vi "Laser Ablation and Capture.vi"() -> ()   [LabVIEW 2016] (continued)
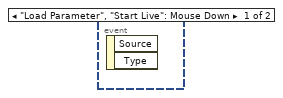
[diagram p2: hidden frame]
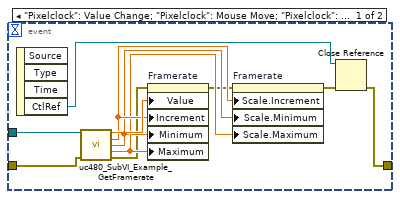
[diagram p3: hidden frame]
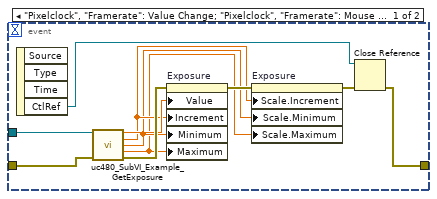
[diagram p4: hidden frame]
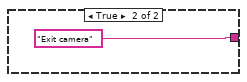
[diagram p5: hidden frame]
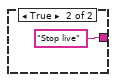
[diagram p6: hidden frame]
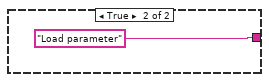
[diagram p7: hidden frame]
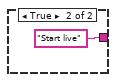
[diagram p8: hidden frame]
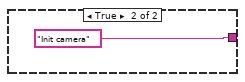
[diagram p9: hidden frame]
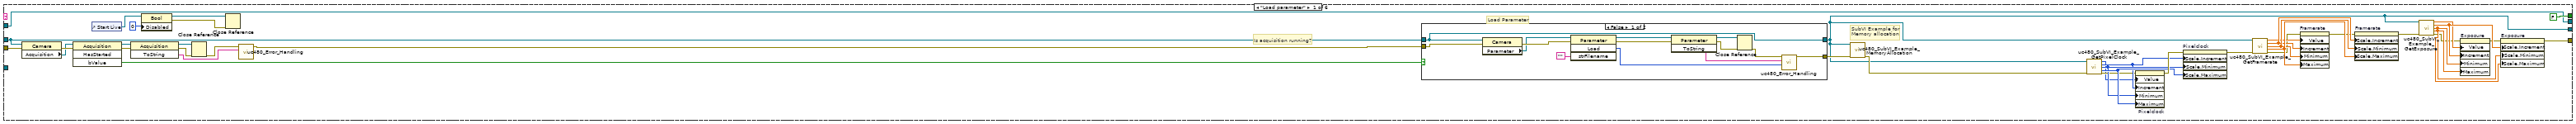
[diagram p10: hidden frame]
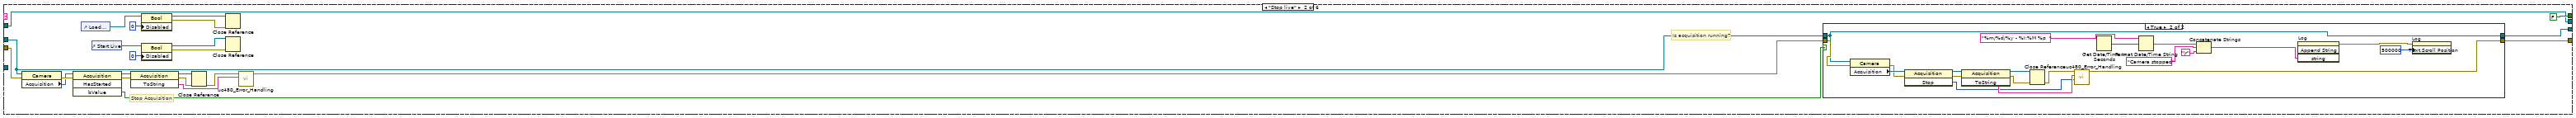
[diagram p12: hidden frame]
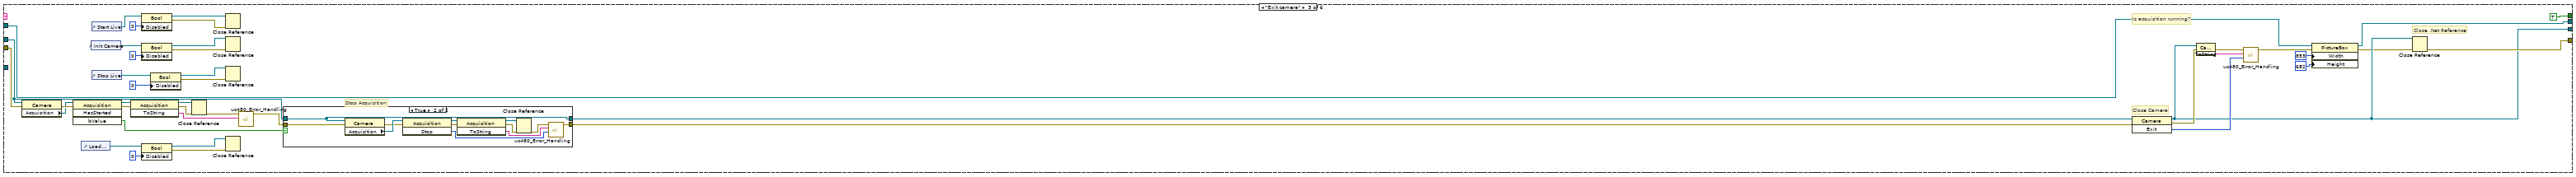
[diagram p14: hidden frame]
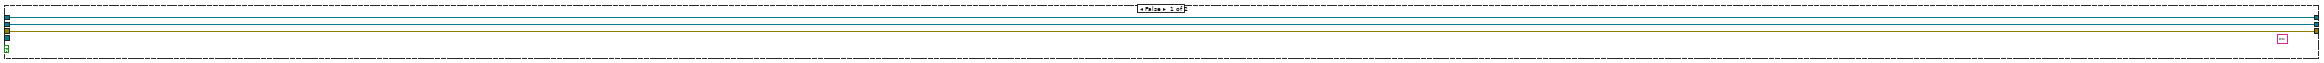
[diagram p16: hidden frame]
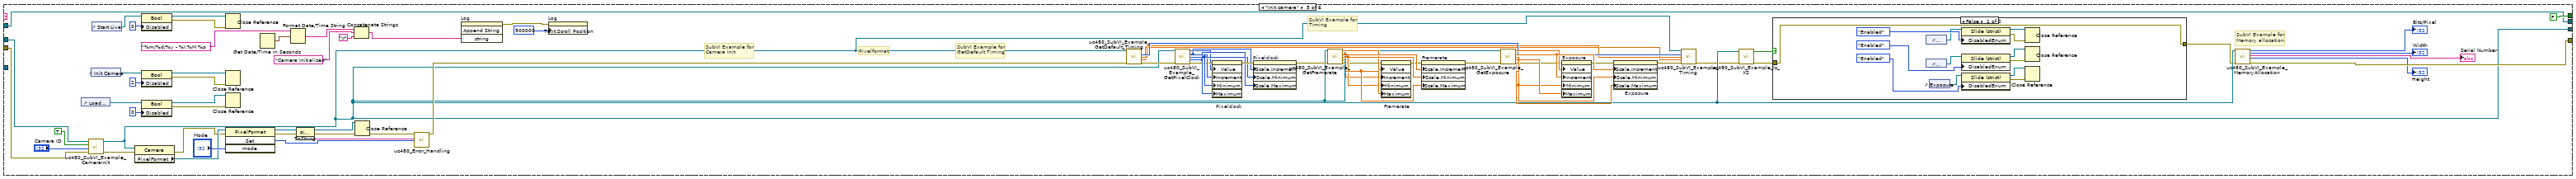
[diagram p18: hidden frame]
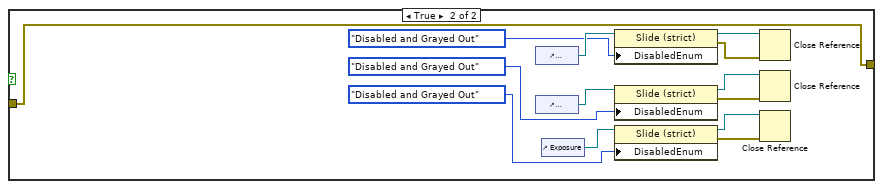
[diagram p19: hidden frame]
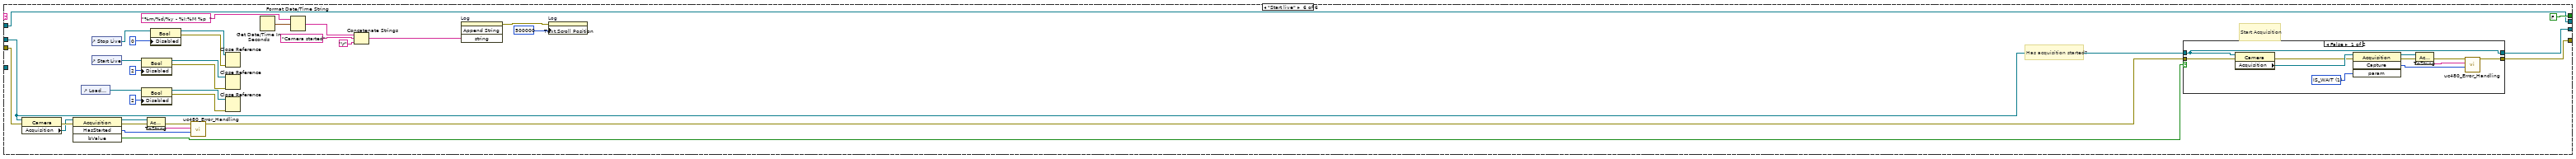
[diagram p20: hidden frame]
            n601 = call <vilib>:"Check if File or Folder Exists.vi"("path"=w1489) -> ("file or folder exists?"=w1488:bool, "dup path"=w1487:path)  [unwired: 8 in, 1 out]
            n602 = case shown="True" w1488 {
              tunnel: w1487 -> [w1499 w1500]
              tunnel: [w1498 w1500] -> w1486
              frame False {
                n603 = Create Folder(path (use dialog)=w1499) -> (created path=w1498:path)  [unwired: 2 in, 2 out]
              }
              frame True {
              }
            }
            n604 = Get Date/Time In Seconds() -> (seconds since 1Jan1904=w1483:timestamp)
            n605 = Format Date/Time String(time format string (%c)="%d%m%y %I-%M %p ", seconds (now)=w1483) -> (date/time string=w1482:string)  [unwired: 1 in]
            n606 = Concatenate Strings(w1482, " - saved ROI.tiff" ("string")) -> (w1480:string)
            n607 = Build Path(base path=w1486, name or relative path=w1480) -> (appended path=w1485:path)
            n608 = call-poly "IMAQ Write File 2"("File Path"=w1485, "Image"=w1493) -> ()  [unwired: 8 in, 2 out]
          }
        }
      }
      event "Load ROI": Value Change {
        n609 = event-data() -> ()  [unwired: 1 in, 6 out]
        n610 = case shown="True" "Load ROI" {
          frame False {
          }
          frame True {
            n611 = call "File Dialog"("prompt"="Select an ROI file..." ("pattern label"), "pattern (all files)"="*.jpg;*.bmp;*.jpeg;*.tif;*.tiff;*.png", "pattern label"="ROI files") -> ("selected path"=w1502:path, "cancelled"=w1503:bool)  [unwired: 9 in, 2 out]
            n612 = case shown="False" w1503 {
              tunnel: w1502 -> [w1514 _]
              frame False {
                n613 = call "IMAQ Create"("Image Name"="untitled") -> ("New Image"=w1516:T2)  [unwired: 4 in, 1 out]
                n614 = call "IMAQ ReadFile"("File Path"=w1514, "Image"=w1516) -> ("Image Out"=w1515:T2)  [unwired: 5 in, 4 out]
                n615 = call "IMAQ MaskToROI"("Image"=w1515) -> ("ROI Descriptor"=w1507:T13)  [unwired: 6 in, 2 out]
                n616 = Unbundle By Name(w1507) -> ("Contours"=w1512:T14)  [unwired: 1 out]
                n617 = Index Array(array=w1512) -> (element=w1513:T15)  [unwired: 1 in]
                n618 = Bundle By Name(cluster=w1513, "Type"=u32 6) -> (w1511:T15)
                n619 = Replace Array Subset(array=w1512, new element=w1511) -> (w1510:T14)  [unwired: 1 in]
                n620 = Bundle By Name(cluster=w1507, "Contours"=w1510) -> (w1508:T13)
                n621 = property on="Source" class="ImageControl"("ROI"=w1508) -> ()  [unwired: 2 in, 2 out]
              }
              frame True {
              }
            }
          }
        }
      }
      event "Axes Manual Control": Value Change {
        n622 = event-data() -> ()  [unwired: 1 in, 6 out]
        n623 = case shown="True" "Axes Manual Control" {
          tunnel: w1520 -> [_ w1532]
          tunnel: w1519 -> [_ w1531]
          tunnel: w1518 -> [_ w1530]
          frame False {
          }
          frame True {
            n624 = flat-sequence {
              tunnel: w1532 -> [w1542]
              tunnel: w1531 -> [w1541]
              tunnel: w1530 -> [w1540]
              tunnel: [w1542] -> w1529
              tunnel: [w1541] -> w1528
              tunnel: [w1540] -> w1527
              tunnel: [w1539] -> w1526
              tunnel: [w1538] -> w1525
              tunnel: [w1537] -> w1524
              tunnel: [w1536] -> w1523
              tunnel: w1529 -> [w1585]
              tunnel: w1528 -> [w1584]
              tunnel: w1527 -> [w1583]
              tunnel: w1526 -> [w1578]
              tunnel: w1525 -> [w1577]
              tunnel: w1524 -> [w1568]
              tunnel: w1523 -> [w1567]
              frame #0 {
                n625 = call <userlib>:"Open TCP-IP.vi"("IP address"=w1542) -> ("error out"=w1534:errorcluster, "Connection ID"=w1543:T9)  [unwired: 8 in, 1 out]
                n626 = call <vilib>:"Simple Error Handler.vi"("error in (no error)"=w1534) -> ("error?"=w1533:bool, "error out"=w1535:errorcluster)  [unwired: 4 in, 3 out]
                n627 = case shown="True" w1533 {
                  tunnel: w1543 -> [w1558 _]
                  tunnel: w1535 -> [w1557 _]
                  tunnel: w1541 -> [w1554 _]
                  tunnel: w1540 -> [w1553 _]
                  tunnel: [w1552 w1562] -> w1539
                  tunnel: [w1551 w1562] -> w1538
                  tunnel: [w1547 w1561] -> w1537
                  tunnel: [w1546 w1561] -> w1536
                  frame False {
                    n628 = call "Get Stages Status.vi"("error in (no error)"=w1557, "Group Name (250 c max)"=w1554, "connection ID in"=w1558) -> ("error out"=w1556:errorcluster, "XPS error out"=w1555:errorcluster, "Group Status String"=w1551:string, "connection ID out"=w1550:T9, "Status"=w1546:i32)  [unwired: 4 in]
                    n629 = call "Get Stages Status.vi"("error in (no error)"=w1556, "XPS error in (no error)"=w1555, "Group Name (250 c max)"=w1553, "connection ID in"=w1550) -> ("error out"=w1560:errorcluster, "XPS error out"=w1549:errorcluster, "Group Status String"=w1552:string, "connection ID out"=w1559:T9, "Status"=w1547:i32)  [unwired: 3 in]
                    n630 = call <vilib>:"Simple Error Handler.vi"("error source (\" \")"="Axis manual control check" ("error source (\" \")"), "error in (no error)"=w1549) -> ()  [unwired: 3 in, 5 out]
                    n631 = call <userlib>:"Close TCP-IP.vi"("error in (no error)"=w1560, "connection ID in"=w1559) -> ("Error out"=w1548:errorcluster)  [unwired: 9 in]
                    n632 = call <vilib>:"Simple Error Handler.vi"("error source (\" \")"="TCP close Axis manual control check" ("error source (\" \")"), "error in (no error)"=w1548) -> ()  [unwired: 3 in, 5 out]
                  }
                  frame True {
                    w1561 = 0
                    w1562 = ""
                  }
                }
              }
              frame #1 {
                w1571 = 47 ("y")
                w1572 = "Ready"
                n633 = String Subset(string=w1577, offset (0)=0, length (rest)=5 ("length (rest)")) -> (substring=w1574:string)
                n634 = String Subset(string=w1578, offset (0)=0, length (rest)=5 ("length (rest)")) -> (substring=w1573:string)
                n635 = Equal?(x=w1574, y=w1572) -> (x = y?=w1575:bool)
                n636 = Equal?(x=w1572, y=w1573) -> (x = y?=w1576:bool)
                n637 = Equal?(x=w1571, y=w1567) -> (x = y?=w1569:bool)
                n638 = Equal?(x=w1568, y=w1571) -> (x = y?=w1570:bool)
                n639 = And(x=w1570, y=w1569) -> (x .and. y?=w1564:bool)
                n640 = And(x=w1575, y=w1576) -> (x .and. y?=w1565:bool)
                n641 = Not(x=w1564) -> (.not. x?=w1563:bool)
                n642 = And(x=w1565, y=w1563) -> (x .and. y?=w1566:bool)
                n643 = case shown="True" w1566 {
                  tunnel: w1585 -> [_ w1593]
                  tunnel: w1584 -> [_ w1592]
                  tunnel: w1583 -> [_ w1591]
                  tunnel: w1563 -> [w1586 _]
                  frame False {
                    n644 = case shown="False" w1586 {
                      frame False {
                        n645 = One Button Dialog(message="One or more axis already in jogging position") -> ()  [unwired: 1 in, 1 out]
                      }
                      frame True {
                        n646 = One Button Dialog(message="Axes are not ready") -> ()  [unwired: 1 in, 1 out]
                      }
                    }
                  }
                  frame True {
                    n647 = local read "Axis 2 inverted?"() -> (w1590:bool)
                    n648 = local read "Axis 1 inverted?"() -> (w1589:bool)
                    n649 = call "XPS Controller.vi"("Axis 2"=w1591, "Axis 1"=w1592, "Controller Address"=w1593, "Axis 2 \ninverted?"=w1590, "Axis 1 \ninverted?"=w1589) -> ()  [unwired: 6 in]
                  }
                }
              }
            }
          }
        }
      }
      event "Home Axes": Value Change {
        n650 = event-data() -> ()  [unwired: 1 in, 6 out]
        n651 = flat-sequence {
          tunnel: w1600 -> [w1606]
          tunnel: w1601 -> [w1607]
          tunnel: w1602 -> [w1608]
          tunnel: "Home Axes" -> [w1609]
          tunnel: [w1609] -> w1598
          tunnel: [w1608] -> w1597
          tunnel: [w1607] -> w1596
          tunnel: [w1606] -> w1595
          tunnel: [w1605] -> w1594
          tunnel: [w1613] -> w1599
          tunnel: w1598 -> [w1611]
          tunnel: w1597 -> [w1616]
          tunnel: w1596 -> [w1614]
          tunnel: w1595 -> [w1615]
          tunnel: w1594 -> [w1612]
          tunnel: [w1695] -> w1603
          tunnel: w1599 -> [w1694]
          frame #0 {
            n652 = call "Display Message to User"() -> ("OK"=w1605:bool)  [unwired: 10 in, 1 out]
          }
          frame #1 {
            n653 = And(x=w1611, y=w1612) -> (x .and. y?=w1610:bool)
            n654 = case shown="True" w1610 {
              tunnel: w1616 -> [_ w1632]
              tunnel: w1614 -> [_ w1633]
              tunnel: w1615 -> [_ w1630]
              tunnel: w1614 -> [_ w1631]
              tunnel: [FALSE w1623] -> w1613
              frame False {
              }
              frame True {
                w1629 = 47 ("y")
                w1645 = "Ready"
                n655 = call <userlib>:"Open TCP-IP.vi"("IP address"=w1632) -> ("error out"=w1618:errorcluster, "Connection ID"=w1636:T9)  [unwired: 8 in, 1 out]
                n656 = call <vilib>:"Simple Error Handler.vi"("error in (no error)"=w1618) -> ("error?"=w1620:bool, "error out"=w1619:errorcluster)  [unwired: 4 in, 3 out]
                n657 = case shown="False" w1620 {
                  tunnel: w1619 -> [w1659 _]
                  tunnel: w1636 -> [w1658 _]
                  tunnel: [w1655 w1664] -> w1635
                  tunnel: [w1654 w1664] -> w1634
                  tunnel: w1633 -> [w1653 _]
                  tunnel: w1630 -> [w1652 _]
                  tunnel: [w1649 w1663] -> w1628
                  tunnel: [w1648 w1663] -> w1627
                  frame False {
                    n658 = call "Get Stages Status.vi"("error in (no error)"=w1659, "Group Name (250 c max)"=w1653, "connection ID in"=w1658) -> ("error out"=w1660:errorcluster, "XPS error out"=w1661:errorcluster, "Group Status String"=w1655:string, "connection ID out"=w1662:T9, "Status"=w1648:i32)  [unwired: 4 in]
                    n659 = call "Get Stages Status.vi"("error in (no error)"=w1660, "XPS error in (no error)"=w1661, "Group Name (250 c max)"=w1652, "connection ID in"=w1662) -> ("error out"=w1656:errorcluster, "XPS error out"=w1651:errorcluster, "Group Status String"=w1654:string, "connection ID out"=w1657:T9, "Status"=w1649:i32)  [unwired: 3 in]
                    n660 = call <vilib>:"Simple Error Handler.vi"("error source (\" \")"="home axis check" ("error source (\" \")"), "error in (no error)"=w1651) -> ()  [unwired: 3 in, 5 out]
                    n661 = call <userlib>:"Close TCP-IP.vi"("error in (no error)"=w1656, "connection ID in"=w1657) -> ("Error out"=w1650:errorcluster)  [unwired: 9 in]
                    n662 = call <vilib>:"Simple Error Handler.vi"("error source (\" \")"="TCP close home axis check" ("error source (\" \")"), "error in (no error)"=w1650) -> ()  [unwired: 3 in, 5 out]
                  }
                  frame True {
                    w1663 = 0
                    w1664 = ""
                  }
                }
                n663 = Equal?(x=w1629, y=w1627) -> (x = y?=w1626:bool)
                n664 = Equal?(x=w1628, y=w1629) -> (x = y?=w1625:bool)
                n665 = String Subset(string=w1635, offset (0)=0, length (rest)=5 ("length (rest)")) -> (substring=w1643:string)
                n666 = String Subset(string=w1634, offset (0)=0, length (rest)=5 ("length (rest)")) -> (substring=w1644:string)
                n667 = Equal?(x=w1643, y=w1645) -> (x = y?=w1642:bool)
                n668 = Equal?(x=w1645, y=w1644) -> (x = y?=w1641:bool)
                n669 = And(x=w1625, y=w1626) -> (x .and. y?=w1621:bool)
                n670 = Not(x=w1621) -> (.not. x?=w1622:bool)
                n671 = And(x=w1642, y=w1641) -> (x .and. y?=w1624:bool)
                n672 = And(x=w1624, y=w1622) -> (x .and. y?=w1623:bool)
                n673 = case shown="True" w1623 {
                  tunnel: w1632 -> [_ w1674]
                  tunnel: w1631 -> [_ w1673]
                  tunnel: w1630 -> [_ w1672]
                  tunnel: w1621 -> [w1665 _]
                  frame False {
                    n674 = case shown="True" w1665 {
                      frame False {
                        n675 = One Button Dialog(message="Axes are not ready") -> ()  [unwired: 1 in, 1 out]
                      }
                      frame True {
                        n676 = One Button Dialog(message="One or more axis are in jogging mode") -> ()  [unwired: 1 in, 1 out]
                      }
                    }
                  }
                  frame True {
                    n677 = call <userlib>:"Open TCP-IP.vi"("IP address"=w1674) -> ("error out"=w1690:errorcluster, "Connection ID"=w1691:T9)  [unwired: 8 in, 1 out]
                    n678 = call <userlib>:"Group Kill.vi"("error in (no error)"=w1690, "Group Name (250 c max)"=w1673, "connection ID in"=w1691) -> ("error out"=w1688:errorcluster, "XPS error out"=w1689:errorcluster, "connection ID out"=w1685:T9)  [unwired: 6 in]
                    n679 = call <userlib>:"Group Initialize.vi"("error in (no error)"=w1688, "XPS error in (no error)"=w1689, "Group Name (250 c max)"=w1673, "connection ID in"=w1685) -> ("error out"=w1686:errorcluster, "XPS error out"=w1687:errorcluster, "connection ID out"=w1684:T9)  [unwired: 5 in]
                    n680 = call <userlib>:"Group Home Search.vi"("error in (no error)"=w1686, "XPS error in (no error)"=w1687, "Group Name (250 c max)"=w1673, "connection ID in"=w1684) -> ("error out"=w1675:errorcluster, "XPS error out"=w1676:errorcluster, "connection ID out"=w1683:T9)  [unwired: 5 in]
                    n681 = call <userlib>:"Group Kill.vi"("error in (no error)"=w1675, "XPS error in (no error)"=w1676, "Group Name (250 c max)"=w1672, "connection ID in"=w1683) -> ("error out"=w1677:errorcluster, "XPS error out"=w1678:errorcluster, "connection ID out"=w1682:T9)  [unwired: 5 in]
                    n682 = call <userlib>:"Group Initialize.vi"("error in (no error)"=w1677, "XPS error in (no error)"=w1678, "Group Name (250 c max)"=w1672, "connection ID in"=w1682) -> ("error out"=w1679:errorcluster, "XPS error out"=w1680:errorcluster, "connection ID out"=w1681:T9)  [unwired: 5 in]
                    n683 = call <userlib>:"Group Home Search.vi"("error in (no error)"=w1679, "XPS error in (no error)"=w1680, "Group Name (250 c max)"=w1672, "connection ID in"=w1681) -> ("error out"=w1692:errorcluster, "XPS error out"=w1671:errorcluster, "connection ID out"=w1693:T9)  [unwired: 5 in]
                    n684 = call <vilib>:"Simple Error Handler.vi"("error source (\" \")"="home axis " ("error source (\" \")"), "error in (no error)"=w1671) -> ()  [unwired: 3 in, 5 out]
                    n685 = call <userlib>:"Close TCP-IP.vi"("error in (no error)"=w1692, "connection ID in"=w1693) -> ("Error out"=w1670:errorcluster)  [unwired: 9 in]
                    n686 = call <vilib>:"Simple Error Handler.vi"("error source (\" \")"="TCP close home axis " ("error source (\" \")"), "error in (no error)"=w1670) -> ()  [unwired: 3 in, 5 out]
                  }
                }
              }
            }
          }
          frame #2 {
            n687 = case shown="True" w1694 {
              tunnel: ["" ("StringOut") "Axes have been moved to home position" ("StringOut")] -> w1695
              frame False {
              }
              frame True {
              }
            }
          }
        }
      }
      event "Transparency": Value Change {
        n688 = event-data() -> ()  [unwired: 1 in, 6 out]
        n689 = control-ref of="This VI"() -> (w1699:refnum<vi>)
        n690 = property class="VI"(reference=w1699, "FP:Transparency"="Transparency") -> ()  [unwired: 1 in, 2 out]
      }
      event "Capture": Value Change {
        w1700 = 47 ("y")
        w1726 = "Ready"
        n691 = event-data() -> ()  [unwired: 1 in, 6 out]
        n692 = call <userlib>:"Open TCP-IP.vi"("IP address"=w1714) -> ("error out"=w1703:errorcluster, "Connection ID"=w1717:T9)  [unwired: 8 in, 1 out]
        n693 = call <vilib>:"Simple Error Handler.vi"("error in (no error)"=w1703) -> ("error?"=w1701:bool, "error out"=w1702:errorcluster)  [unwired: 4 in, 3 out]
        n694 = case shown="False" w1701 {
          tunnel: w1702 -> [w1740 _]
          tunnel: w1717 -> [w1739 _]
          tunnel: [w1736 w1744] -> w1716
          tunnel: [w1735 w1744] -> w1715
          tunnel: w1713 -> [w1734 _]
          tunnel: w1712 -> [w1733 _]
          tunnel: [w1731 w1745] -> w1711
          tunnel: [w1730 w1745] -> w1710
          frame False {
            n695 = call "Get Stages Status.vi"("error in (no error)"=w1740, "Group Name (250 c max)"=w1734, "connection ID in"=w1739) -> ("error out"=w1741:errorcluster, "XPS error out"=w1742:errorcluster, "Group Status String"=w1736:string, "connection ID out"=w1743:T9, "Status"=w1730:i32)  [unwired: 4 in]
            n696 = call "Get Stages Status.vi"("error in (no error)"=w1741, "XPS error in (no error)"=w1742, "Group Name (250 c max)"=w1733, "connection ID in"=w1743) -> ("error out"=w1737:errorcluster, "XPS error out"=w1732:errorcluster, "Group Status String"=w1735:string, "connection ID out"=w1738:T9, "Status"=w1731:i32)  [unwired: 3 in]
            n697 = call <vilib>:"Simple Error Handler.vi"("error source (\" \")"="Capture check" ("error source (\" \")"), "error in (no error)"=w1732) -> ()  [unwired: 3 in, 5 out]
            n698 = call <userlib>:"Close TCP-IP.vi"("error in (no error)"=w1737, "connection ID in"=w1738) -> ("Error out"=w1728:errorcluster)  [unwired: 9 in]
            n699 = call <vilib>:"Simple Error Handler.vi"("error in (no error)"=w1728) -> ()  [unwired: 4 in, 5 out]
          }
          frame True {
            w1745 = 0
            w1744 = ""
          }
        }
        n700 = Equal?(x=w1711, y=w1700) -> (x = y?=w1709:bool)
        n701 = Equal?(x=w1700, y=w1710) -> (x = y?=w1708:bool)
        n702 = String Subset(string=w1716, offset (0)=0, length (rest)=5 ("length (rest)")) -> (substring=w1724:string)
        n703 = String Subset(string=w1715, offset (0)=0, length (rest)=5 ("length (rest)")) -> (substring=w1725:string)
        n704 = Equal?(x=w1724, y=w1726) -> (x = y?=w1723:bool)
        n705 = Equal?(x=w1726, y=w1725) -> (x = y?=w1722:bool)
        n706 = And(x=w1709, y=w1708) -> (x .and. y?=w1705:bool)
        n707 = Not(x=w1705) -> (.not. x?=w1704:bool)
        n708 = And(x=w1723, y=w1722) -> (x .and. y?=w1707:bool)
        n709 = And(x=w1707, y=w1704) -> (x .and. y?=w1706:bool)
        n710 = case shown="True" w1706 {
          tunnel: ["" w1771] -> w1727
          tunnel: w1714 -> [_ w1770]
          tunnel: w1712 -> [_ w1769]
          tunnel: w1713 -> [_ w1768]
          tunnel: w1705 -> [w1746 _]
          frame False {
            n711 = case shown="True" w1746 {
              frame False {
                n712 = One Button Dialog(message="Axes are not ready") -> ()  [unwired: 1 in, 1 out]
              }
              frame True {
                n713 = One Button Dialog(message="One or more axis are in jogging mode") -> ()  [unwired: 1 in, 1 out]
              }
            }
          }
          frame True {
            n714 = flat-sequence {
              tunnel: [w1801] -> w1782
              tunnel: [w1787] -> w1781
              tunnel: [w1786] -> w1780
              tunnel: [w1800] -> w1779
              tunnel: [w1799] -> w1778
              tunnel: [w1798] -> w1777
              tunnel: [w1785] -> w1776
              tunnel: w1768 -> [w1796]
              tunnel: w1769 -> [w1797]
              tunnel: w1770 -> [w1785]
              tunnel: [w1784] -> w1757
              tunnel: [w1783] -> w1753
              tunnel: w1782 -> [w1821]
              tunnel: w1781 -> [w1809]
              tunnel: w1780 -> [w1808]
              tunnel: w1779 -> [w1819]
              tunnel: w1778 -> [w1818]
              tunnel: [w1813] -> w1775
              tunnel: w1777 -> [w1813]
              tunnel: [w1812] -> w1774
              tunnel: w1776 -> [w1812]
              tunnel: [w1809] -> w1767
              tunnel: [w1808] -> w1765
              tunnel: [w1807] -> w1758
              tunnel: w1757 -> [w1807]
              tunnel: [w1806] -> w1754
              tunnel: w1753 -> [w1806]
              tunnel: [w1827] -> w1773
              tunnel: w1775 -> [w1827]
              tunnel: [w1826] -> w1772
              tunnel: w1774 -> [w1826]
              tunnel: w1767 -> [w1825]
              tunnel: [w1825] -> w1766
              tunnel: w1765 -> [w1824]
              tunnel: [w1824] -> w1764
              tunnel: [w1823] -> w1759
              tunnel: w1758 -> [w1823]
              tunnel: [w1822] -> w1755
              tunnel: w1754 -> [w1822]
              tunnel: w1773 -> [w1841]
              tunnel: w1772 -> [w1831]
              tunnel: [w1840] -> w1763
              tunnel: w1766 -> [w1830]
              tunnel: w1764 -> [w1829]
              tunnel: [w1834] -> w1761
              tunnel: [w1833] -> w1760
              tunnel: w1759 -> [w1833]
              tunnel: [w1832] -> w1756
              tunnel: w1755 -> [w1832]
              tunnel: [w1831] -> w1752
              tunnel: [w1830] -> w1751
              tunnel: [w1829] -> w1750
              tunnel: w1763 -> [w1863]
              tunnel: [w1863] -> w1762
              tunnel: w1761 -> [w1859]
              tunnel: w1760 -> [w1853]
              tunnel: w1756 -> [w1852]
              tunnel: w1752 -> [w1857]
              tunnel: w1751 -> [w1851]
              tunnel: w1750 -> [w1850]
              tunnel: [w1868] -> w1771
              tunnel: w1762 -> [w1865]
              frame #0 {
                w1805 = ".Pos"
                n715 = call <userlib>:"Open TCP-IP.vi"("IP address"=w1785) -> ("error out"=w1790:errorcluster, "Connection ID"=w1792:T9)  [unwired: 5 in, 4 out]
                n716 = Concatenate Strings(w1797, w1805) -> (w1786:string)
                n717 = Concatenate Strings(w1796, w1805) -> (w1787:string)
                n718 = call <userlib>:"Single Axis Group Position Current Get.vi"("error in (no error)"=w1790, "SingleAxis Group  Name (250 c max)"=w1787, "connection ID in"=w1792) -> ("error out"=w1793:errorcluster, "XPS error out"=w1794:errorcluster, "Current Position (units)"=w1783:dbl, "connection ID out"=w1795:T9)  [unwired: 5 in]
                "Pre-Capture Axis 1" <- w1783
                n719 = call <userlib>:"Single Axis Group Position Current Get.vi"("error in (no error)"=w1793, "XPS error in (no error)"=w1794, "SingleAxis Group  Name (250 c max)"=w1786, "connection ID in"=w1795) -> ("error out"=w1789:errorcluster, "XPS error out"=w1788:errorcluster, "Current Position (units)"=w1784:dbl, "connection ID out"=w1791:T9)  [unwired: 4 in]
                "Pre-Capture Axis 2" <- w1784
                n720 = local read "Axis Initial Parameters"() -> (w1798:T1)
                n721 = call <userlib>:"Positioner SGamma Parameters Set.vi"("SGamma Parameters"=w1798, "error in (no error)"=w1789, "XPS error in (no error)"=w1788, "Positioner Name (250 c max)"=w1787, "connection ID in"=w1791) -> ("error out"=w1802:errorcluster, "XPS error out"=w1803:errorcluster, "connection ID out"=w1804:T9)  [unwired: 4 in]
                n722 = call <userlib>:"Positioner SGamma Parameters Set.vi"("SGamma Parameters"=w1798, "error in (no error)"=w1802, "XPS error in (no error)"=w1803, "Positioner Name (250 c max)"=w1786, "connection ID in"=w1804) -> ("error out"=w1800:errorcluster, "XPS error out"=w1799:errorcluster, "connection ID out"=w1801:T9)  [unwired: 4 in]
              }
              frame #1 {
                n723 = local read "Axis 1 Offset"() -> (w1811:dbl)
                n724 = local read "Axis 2 Offset"() -> (w1810:dbl)
                n725 = call <userlib>:"Single Axis Group Move Relative.vi"("Target Displacement (units)"=w1811, "error in (no error)"=w1819, "XPS error in (no error)"=w1818, "SingleAxis Group  Name (250 c max)"=w1809, "connection ID in"=w1821) -> ("error out"=w1816:errorcluster, "XPS error out"=w1817:errorcluster, "connection ID out"=w1820:T9)  [unwired: 4 in]
                n726 = call <userlib>:"Single Axis Group Move Relative.vi"("Target Displacement (units)"=w1810, "error in (no error)"=w1816, "XPS error in (no error)"=w1817, "SingleAxis Group  Name (250 c max)"=w1808, "connection ID in"=w1820) -> ("error out"=w1814:errorcluster, "connection ID out"=w1815:T9)  [unwired: 4 in, 1 out]
                n727 = call <userlib>:"Close TCP-IP.vi"("error in (no error)"=w1814, "connection ID in"=w1815) -> ()  [unwired: 9 in, 1 out]
              }
              frame #2 {
                n728 = Wait (ms)(milliseconds to wait=u32 1000) -> ()  [unwired: 1 out]
              }
              frame #3 {
                n729 = local read "Speed (µm/s)"() -> (w1845:i32)
                n730 = local read "Processi time (sec)"() -> (w1839:i32)
                n731 = local read "Laser on/off array"() -> (w1848:bool[][])
                n732 = local read "Commands array"() -> (w1849:string[][])
                n733 = local read "ROI Area \n(mm2)"() -> (w1837:dbl)
                n734 = local read "Laser Com Delay"() -> (w1836:i32)
                n735 = local read "VISA Laser port"() -> (w1835:string)
                n736 = Divide(x=w1845, y=1000) -> (x/y=w1842:dbl)
                n737 = call "Capture.vi"("Commands array"=w1849, "XPS_Address"=w1831, "VISA resource name"=w1835, "laser array index"=0, "Process time"=w1839, "Axis Speed"=w1842, "Laser on/off array"=w1848, "stop"=FALSE ("STOP CAPTURE"), "delay before read (ms)"=w1836, "Axis Initial Parameters"=w1841, "ROI Area \n(mm2)"=w1837, "Axis 2"=w1829, "Axis 1"=w1830, "OPO on?"=TRUE, "Acceleration (units/seconds²)"="Acceleration \n(mm/s²)") -> ("Elapsed time"=w1840:dbl, "XPS error out"=w1834:errorcluster)  [unwired: 2 in, 1 out]
              }
              frame #4 {
                n738 = call <userlib>:"Open TCP-IP.vi"("IP address"=w1857) -> ("error out"=w1856:errorcluster, "Connection ID"=w1858:T9)  [unwired: 5 in, 4 out]
                n739 = call <userlib>:"Single Axis Group Move Absolute.vi"("Target Position (units)"=w1852, "error in (no error)"=w1856, "XPS error in (no error)"=w1859, "SingleAxis Group  Name (250 c max)"=w1851, "connection ID in"=w1858) -> ("error out"=w1861:errorcluster, "XPS error out"=w1860:errorcluster, "connection ID out"=w1862:T9)  [unwired: 4 in]
                n740 = call <userlib>:"Single Axis Group Move Absolute.vi"("Target Position (units)"=w1853, "error in (no error)"=w1861, "XPS error in (no error)"=w1860, "SingleAxis Group  Name (250 c max)"=w1850, "connection ID in"=w1862) -> ("error out"=w1854:errorcluster, "connection ID out"=w1855:T9)  [unwired: 4 in, 1 out]
                n741 = call <userlib>:"Close TCP-IP.vi"("error in (no error)"=w1854, "connection ID in"=w1855) -> ()  [unwired: 9 in, 1 out]
              }
              frame #5 {
                n742 = Number To Decimal String(number=w1865) -> (decimal integer string=w1864:string)  [unwired: 1 in]
                n743 = Concatenate Strings("Capture completed in " ("StringOut"), w1864, " seconds" ("string")) -> (w1868:string)
              }
            }
          }
        }
      }
      event "Microscope/Capture \nstatus button": Value Change {
        w1888 = 47 ("y")
        w1901 = "Ready"
        n744 = event-data() -> ()  [unwired: 1 in, 6 out]
        n745 = call <userlib>:"Open TCP-IP.vi"("IP address"=w1871) -> ("error out"=w1904:errorcluster, "Connection ID"=w1905:T9)  [unwired: 8 in, 1 out]
        n746 = call <vilib>:"Simple Error Handler.vi"("error in (no error)"=w1904) -> ("error?"=w1902:bool, "error out"=w1903:errorcluster)  [unwired: 4 in, 3 out]
        n747 = case shown="False" w1902 {
          tunnel: w1905 -> [w1983 _]
          tunnel: [w1980 w1987] -> w1887
          tunnel: [w1979 w1987] -> w1886
          tunnel: w1881 -> [w1978 _]
          tunnel: w1882 -> [w1977 _]
          tunnel: [w1975 w1988] -> w1885
          tunnel: [w1974 w1988] -> w1884
          tunnel: w1903 -> [w1971 _]
          frame False {
            n748 = call "Get Stages Status.vi"("error in (no error)"=w1971, "Group Name (250 c max)"=w1978, "connection ID in"=w1983) -> ("error out"=w1984:errorcluster, "XPS error out"=w1985:errorcluster, "Group Status String"=w1980:string, "connection ID out"=w1986:T9, "Status"=w1974:i32)  [unwired: 4 in]
            n749 = call "Get Stages Status.vi"("error in (no error)"=w1984, "XPS error in (no error)"=w1985, "Group Name (250 c max)"=w1977, "connection ID in"=w1986) -> ("error out"=w1981:errorcluster, "XPS error out"=w1976:errorcluster, "Group Status String"=w1979:string, "connection ID out"=w1982:T9, "Status"=w1975:i32)  [unwired: 3 in]
            n750 = call <vilib>:"Simple Error Handler.vi"("error source (\" \")"="Axes check" ("error source (\" \")"), "error in (no error)"=w1976) -> ()  [unwired: 3 in, 5 out]
            n751 = call <userlib>:"Close TCP-IP.vi"("error in (no error)"=w1981, "connection ID in"=w1982) -> ("Error out"=w1972:errorcluster)  [unwired: 9 in]
            n752 = call <vilib>:"Simple Error Handler.vi"("error in (no error)"=w1972) -> ()  [unwired: 4 in, 5 out]
          }
          frame True {
            w1988 = 0
            w1987 = ""
          }
        }
        n753 = Equal?(x=w1885, y=w1888) -> (x = y?=w1892:bool)
        n754 = Equal?(x=w1888, y=w1884) -> (x = y?=w1891:bool)
        n755 = String Subset(string=w1887, offset (0)=0, length (rest)=5 ("length (rest)")) -> (substring=w1899:string)
        n756 = String Subset(string=w1886, offset (0)=0, length (rest)=5 ("length (rest)")) -> (substring=w1900:string)
        n757 = case shown="False" "Microscope/Capture \nstatus button" {
          tunnel: ["capture " "microscope "] -> w1875
          frame False {
          }
          frame True {
          }
        }
        n758 = Equal?(x=w1899, y=w1901) -> (x = y?=w1898:bool)
        n759 = Equal?(x=w1901, y=w1900) -> (x = y?=w1897:bool)
        n760 = And(x=w1892, y=w1891) -> (x .and. y?=w1883:bool)
        n761 = Not(x=w1883) -> (.not. x?=w1889:bool)
        n762 = And(x=w1898, y=w1897) -> (x .and. y?=w1890:bool)
        n763 = And(x=w1890, y=w1889) -> (x .and. y?=w1873:bool)
        n764 = Concatenate Strings("Do you want to move the axis to the " ("message"), w1875, "position?" ("string")) -> (w1874:string)
        n765 = Two Button Dialog(message=w1874, 1:"No" ("F button name (\"Cancel\")"), 2:"Yes" ("T button name (\"OK\")")) -> (T button?=w1870:bool)
        n766 = case shown="False" w1870 {
          tunnel: "Microscope/Capture \nstatus button" -> [w1906 _]
          frame False {
            n767 = Not(x=w1906) -> (.not. x?=w1907:bool)
            n768 = local write "Microscope/Capture \nstatus button"(w1907) -> ()
          }
          frame True {
          }
        }
        n769 = And(x=w1873, y=w1870) -> (x .and. y?=w1872:bool)
        n770 = case shown="True" w1872 {
          tunnel: "Microscope/Capture \nstatus button" -> [w1911 w1916]
          tunnel: w1883 -> [w1912 _]
          tunnel: w1882 -> [_ w1924]
          tunnel: w1881 -> [_ w1923]
          tunnel: [_ w1922] -> w1880
          tunnel: w1871 -> [_ w1915]
          frame False {
            n771 = Not(x=w1911) -> (.not. x?=w1910:bool)
            n772 = case shown="True" w1912 {
              frame False {
                n773 = One Button Dialog(message="Axes are not ready") -> ()  [unwired: 1 in, 1 out]
              }
              frame True {
                n774 = One Button Dialog(message="One or more axis are in jogging mode") -> ()  [unwired: 1 in, 1 out]
              }
            }
            n775 = local write "Microscope/Capture \nstatus button"(w1910) -> ()
          }
          frame True {
            n776 = flat-sequence {
              tunnel: [w1935] -> w1921
              tunnel: [w1934] -> w1920
              tunnel: [w1933] -> w1919
              tunnel: [w1932] -> w1918
              tunnel: [w1931] -> w1917
              tunnel: w1924 -> [w1930]
              tunnel: w1923 -> [w1929]
              tunnel: w1915 -> [w1928]
              tunnel: w1921 -> [w1956]
              tunnel: w1920 -> [w1947]
              tunnel: w1919 -> [w1948]
              tunnel: w1918 -> [w1954]
              tunnel: w1917 -> [w1953]
              tunnel: w1916 -> [w1942]
              tunnel: [w1968] -> w1922
              tunnel: w1916 -> [w1964]
              frame #0 {
                w1940 = ".Pos"
                n777 = local read "Axis Initial Parameters"() -> (w1927:T1)
                n778 = Bundle By Name(cluster=w1927, "Velocity (units/seconds)"=10.0) -> (w1925:T1)
                n779 = call <userlib>:"Open TCP-IP.vi"("IP address"=w1928) -> ("error out"=w1936:errorcluster, "Connection ID"=w1941:T9)  [unwired: 5 in, 4 out]
                n780 = Concatenate Strings(w1929, w1940) -> (w1934:string)
                n781 = call <userlib>:"Positioner SGamma Parameters Set.vi"("SGamma Parameters"=w1927, "error in (no error)"=w1936, "Positioner Name (250 c max)"=w1934, "connection ID in"=w1941) -> ("error out"=w1937:errorcluster, "XPS error out"=w1938:errorcluster, "connection ID out"=w1939:T9)  [unwired: 5 in]
                n782 = Concatenate Strings(w1930, w1940) -> (w1933:string)
                n783 = call <userlib>:"Positioner SGamma Parameters Set.vi"("SGamma Parameters"=w1925, "error in (no error)"=w1937, "XPS error in (no error)"=w1938, "Positioner Name (250 c max)"=w1933, "connection ID in"=w1939) -> ("error out"=w1932:errorcluster, "XPS error out"=w1931:errorcluster, "connection ID out"=w1935:T9)  [unwired: 4 in]
              }
              frame #1 {
                n784 = local read "X travel"() -> (w1946:dbl)
                n785 = local read "Y travel"() -> (w1945:dbl)
                n786 = case shown="False" w1942 {
                  tunnel: w1946 -> [w1958 w1962]
                  tunnel: w1945 -> [w1957 w1961]
                  tunnel: [w1957 w1960] -> w1944
                  tunnel: [w1958 w1959] -> w1943
                  frame False {
                  }
                  frame True {
                    n787 = Negate(x=w1962) -> (-x=w1959:dbl)
                    n788 = Negate(x=w1961) -> (-x=w1960:dbl)
                  }
                }
                n789 = call <userlib>:"Single Axis Group Move Relative.vi"("Target Displacement (units)"=w1944, "error in (no error)"=w1954, "XPS error in (no error)"=w1953, "SingleAxis Group  Name (250 c max)"=w1947, "connection ID in"=w1956) -> ("error out"=w1951:errorcluster, "XPS error out"=w1952:errorcluster, "connection ID out"=w1955:T9)  [unwired: 4 in]
                n790 = call <userlib>:"Single Axis Group Move Relative.vi"("Target Displacement (units)"=w1943, "error in (no error)"=w1951, "XPS error in (no error)"=w1952, "SingleAxis Group  Name (250 c max)"=w1948, "connection ID in"=w1955) -> ("error out"=w1949:errorcluster, "connection ID out"=w1950:T9)  [unwired: 4 in, 1 out]
                n791 = call <userlib>:"Close TCP-IP.vi"("error in (no error)"=w1949, "connection ID in"=w1950) -> ()  [unwired: 9 in, 1 out]
              }
              frame #2 {
                n792 = Wait (ms)(milliseconds to wait=u32 1000) -> ()  [unwired: 1 out]
              }
              frame #3 {
                n793 = case shown="True" w1964 {
                  tunnel: ["capture " ("string") "microscope " ("string")] -> w1965
                  frame False {
                  }
                  frame True {
                  }
                }
                n794 = Concatenate Strings("Stages translated to the " ("StringOut"), w1965, "position." ("string")) -> (w1968:string)
              }
            }
          }
        }
      }
    }
    n795 = Get Date/Time In Seconds() -> (seconds since 1Jan1904=w816:timestamp)
    n796 = Format Date/Time String(time format string (%c)="%m/%d/%y - %I:%M %p  ", seconds (now)=w816) -> (date/time string=w815:string)  [unwired: 1 in]
    n797 = Empty String/Path?(string/path=w812) -> (empty?=w814:bool)
    n798 = Concatenate Strings(w815, w812, "\r") -> (w813:string)
    n799 = case shown="False" w814 {
      tunnel: w813 -> [w822 _]
      frame False {
        n800 = invoke on="Log" class="Str" method="Append String"("string"=w822) -> (error out=w821:errorcluster)  [unwired: 3 in, 3 out]
        n801 = property on="Log" class="Str"(error in=w821, "Text.Scroll Position"=u32 500000) -> ()  [unwired: 1 in, 2 out]
      }
      frame True {
      }
    }
  }
  n802 = control-ref of="Init Camera"() -> (w74:refnum<vi>)
  n803 = control-ref of="Stop Live"() -> (w67:refnum<vi>)
  n804 = property class="Bool"(reference=w67, "Disabled"=u8 2 ("Deaktiviert")) -> (reference out=w58:refnum<vi>, error out=w57:errorcluster)  [unwired: 1 in]
  n805 = property class="Bool"(reference=w74, "Disabled"=u8 0 ("Deaktiviert")) -> (reference out=w62:refnum<vi>, error out=w61:errorcluster)  [unwired: 1 in]
  n806 = Close Reference(reference=w58, error in (no error)=w57) -> ()  [unwired: 1 out]
  n807 = Close Reference(reference=w62, error in (no error)=w61) -> ()  [unwired: 1 out]
  n808 = control-ref of="Load Parameter"() -> (w68:refnum<vi>)
  n809 = control-ref of="Start Live"() -> (w71:refnum<vi>)
  n810 = property class="Bool"(reference=w71, "Disabled"=u8 2 ("Deaktiviert")) -> (reference out=w60:refnum<vi>, error out=w59:errorcluster)  [unwired: 1 in]
  n811 = property class="Bool"(reference=w68, "Disabled"=u8 2 ("Deaktiviert")) -> (reference out=w56:refnum<vi>, error out=w55:errorcluster)  [unwired: 1 in]
  n812 = Close Reference(reference=w60, error in (no error)=w59) -> ()  [unwired: 1 out]
  n813 = Close Reference(reference=w56, error in (no error)=w55) -> ()  [unwired: 1 out]
